vi "Derivative of intensity graph V1.2.vi"() -> ()   [LabVIEW 2016] (continued)
  in  "stop viewing ?":bool
  out "Y index 2":dbl=103.0
  in  "Pause viewing ?":bool
  in  "Decimate index":dbl=1.0
  in  "Name":T3={"X"="Vsd (V)", "Y"="VsgL (V)", "Z"="I (A)", "dZ/dX"="dI/dV (S)"}
  in  "Enum":T4(ring)=enum."dz/dx vs x"
  out "Derivative of Data":dbl[][](graph)
  out "Column number":i32=1229
  out "Row number":i32=321
  out "Ex":T5={"Offset"=-0.1923, "Multiplier"=0.0004} {"Offset" format="%#_6p"; "Multiplier" format="%#_6p"}
  in  "Ey":T5={"Offset"=-0.8, "Multiplier"=0.005}
  out "Data":dbl[][](graph)
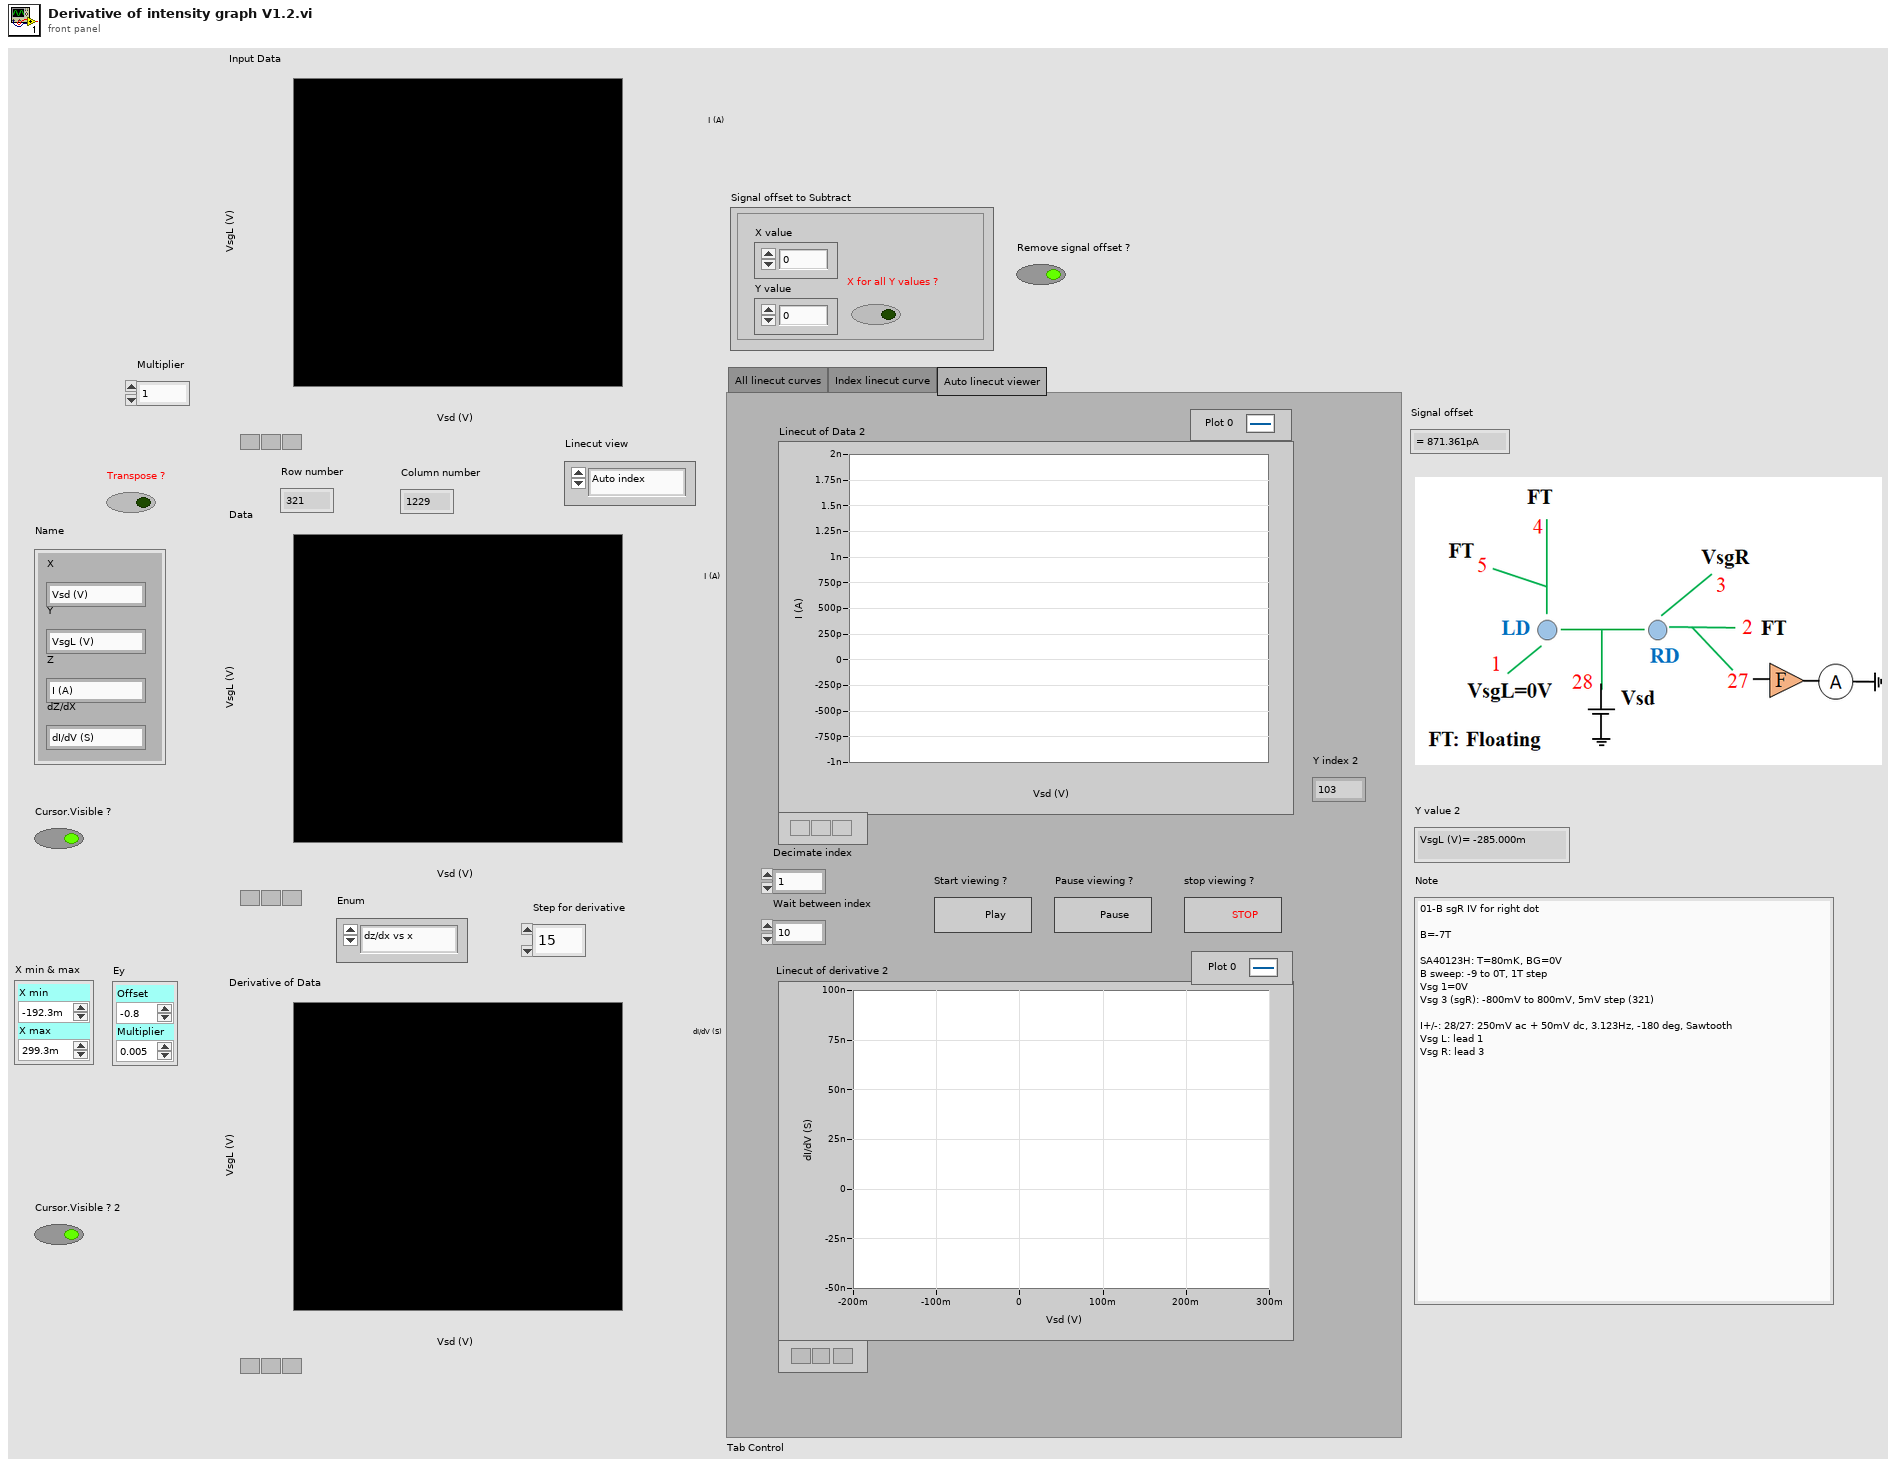
[diagram p1: front panel]
types:
  T1 = cluster{"X value":dbl, "Y value":dbl, "X for all Y values ?":bool}
  T2 = enum32{"All linecut curves", "Index linecut curve", "Auto linecut viewer"}
  T3 = cluster{"X":string, "Y":string, "Z":string, "dZ/dX":string}
  T4 = enum16{"dz/dx vs z", "dz/dx vs x", "dx/dz vs z", "dx/dz vs x"}
  T5 = typedef "LVOffsetAndMultiplierTypeDef.ctl" = cluster{"Offset":dbl, "Multiplier":dbl}
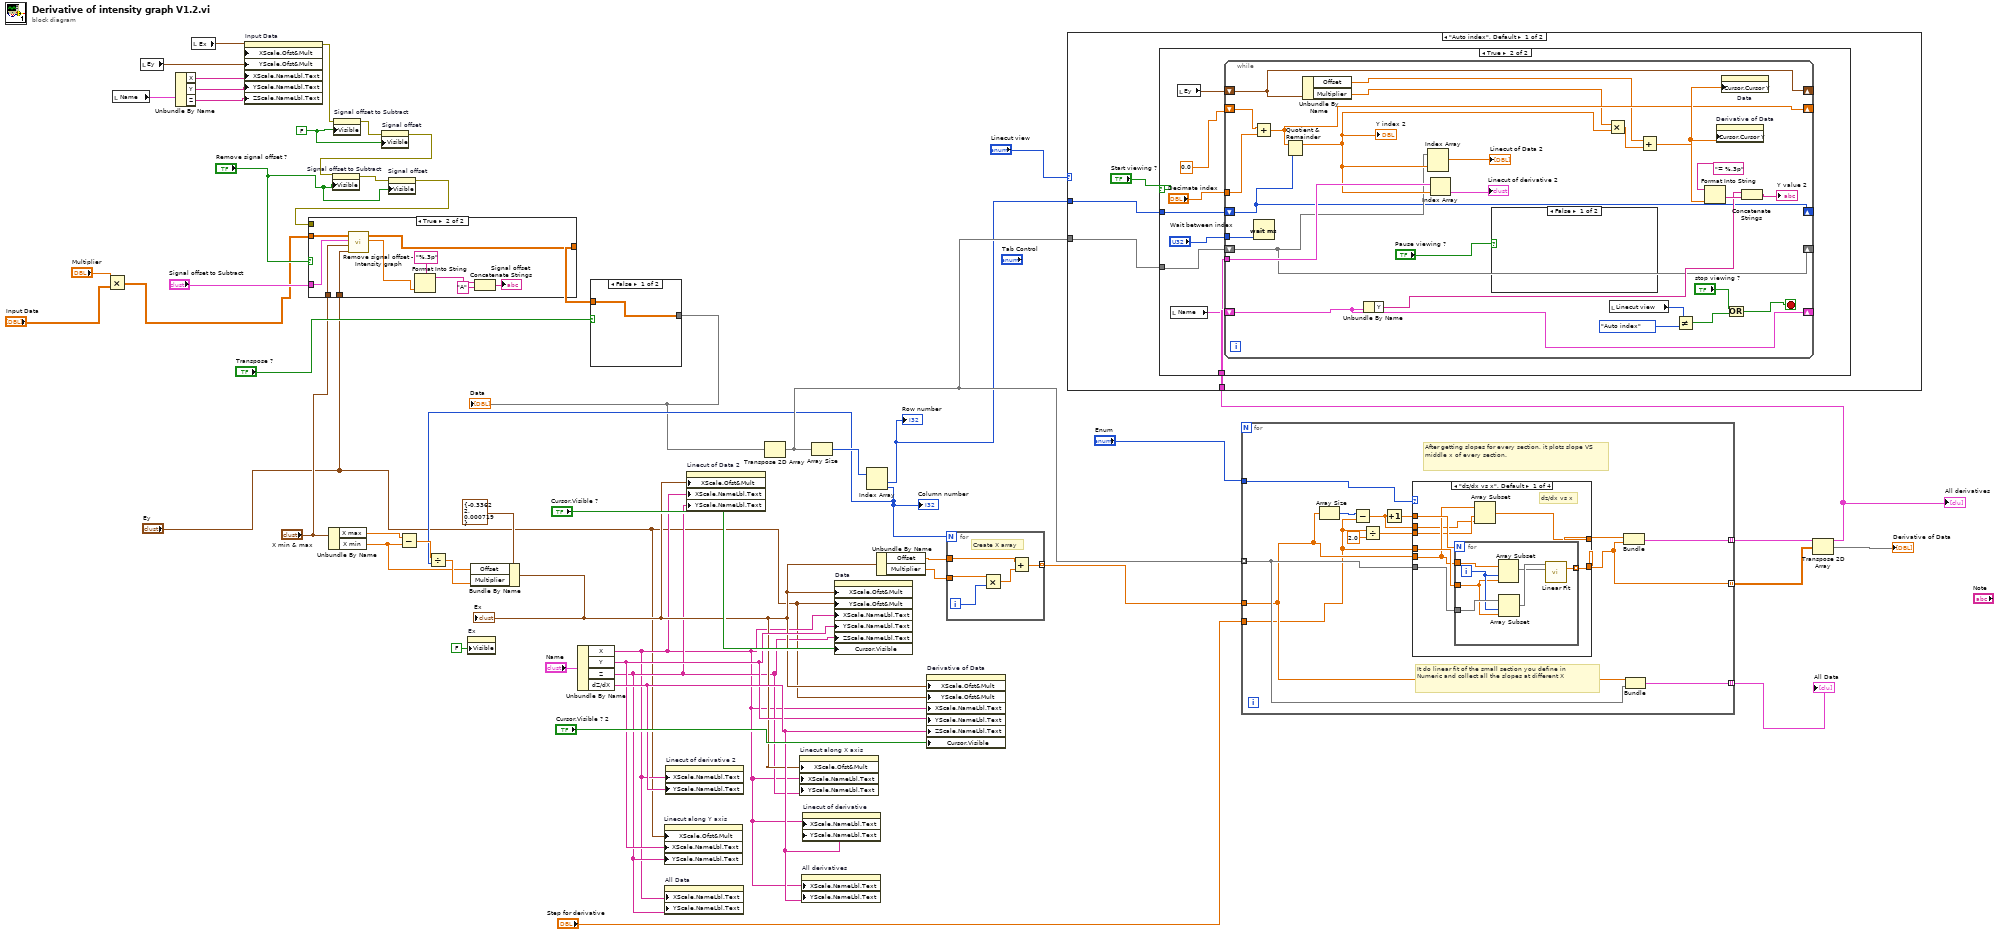
[diagram p0: block diagram]
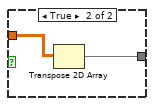
[diagram p3: hidden frame]
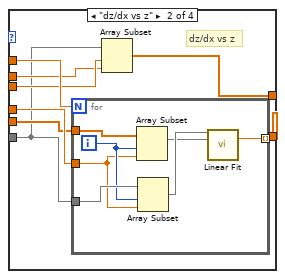
[diagram p4: hidden frame]
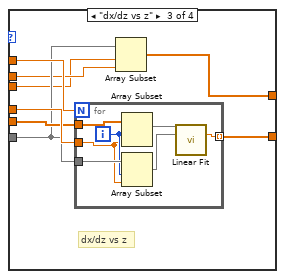
[diagram p5: hidden frame]
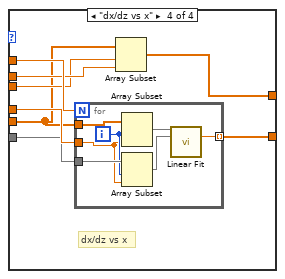
[diagram p6: hidden frame]
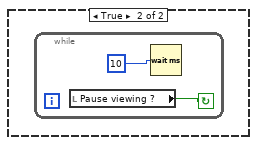
[diagram p8: hidden frame]
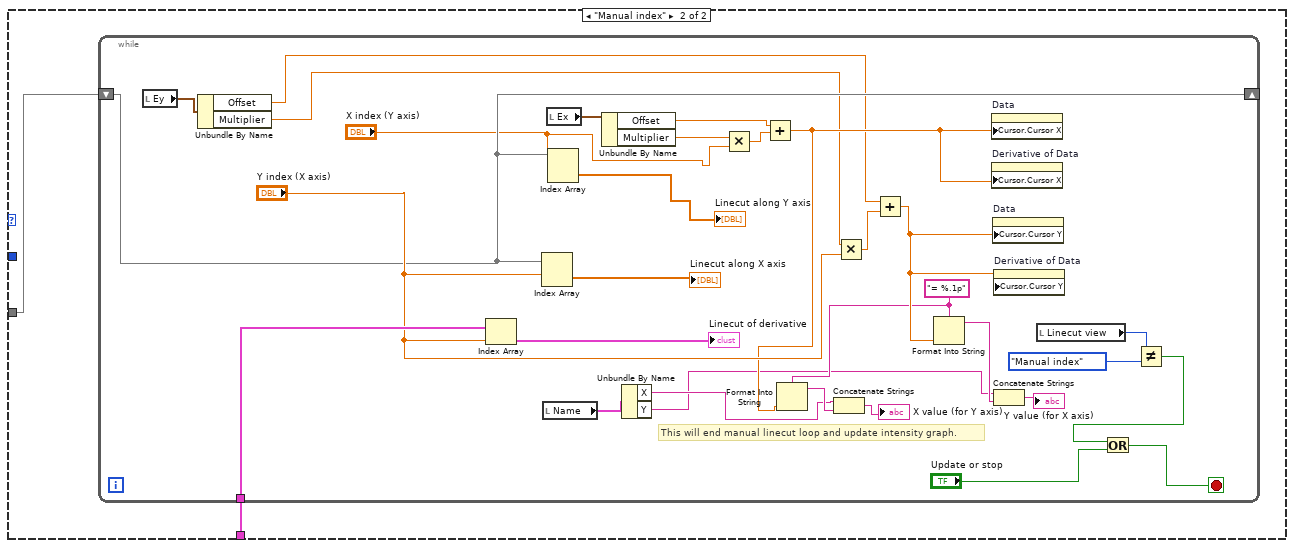
[diagram p9: hidden frame]
diagram:
  w14 = FALSE ("Visible")
  n1 = Multiply(x="Multiplier", y="Input Data") -> (x*y=w3:dbl[][])
  n2 = local read "Name"() -> (w19:T3)
  n3 = local read "Ey"() -> (w8:T5)
  n4 = Unbundle By Name(w19) -> ("X"=w18:string, "Y"=w17:string, "Z"=w16:string)
  n5 = local read "Ex"() -> (w7:T5)
  n6 = property on="Input Data" class="IntGraph (strict)"("XScale.Ofst&Mult"=w7, "YScale.Ofst&Mult"=w8, "XScale.NameLbl.Text"=w18, "YScale.NameLbl.Text"=w17, "ZScale.NameLbl.Text"=w16) -> (error out=w15:errorcluster)  [unwired: 2 in, 1 out]
  n7 = Unbundle By Name("X min & max") -> ("X max"=w32:dbl, "X min"=w27:dbl)
  n8 = property on="Signal offset to Subtract" class="Clust (strict)"(error in=w15, "Visible"=w14) -> (error out=w13:errorcluster)  [unwired: 1 in, 1 out]
  n9 = property on="Signal offset" class="Str"(error in=w13, "Visible"=w14) -> (error out=w12:errorcluster)  [unwired: 1 in, 1 out]
  n10 = property on="Signal offset to Subtract" class="Clust (strict)"(error in=w12, "Visible"="Remove signal offset ?") -> (error out=w10:errorcluster)  [unwired: 1 in, 1 out]
  n11 = property on="Signal offset" class="Str"(error in=w10, "Visible"="Remove signal offset ?") -> (error out=w9:errorcluster)  [unwired: 1 in, 1 out]
  n12 = case shown="True" "Remove signal offset ?" {
    tunnel: w3 -> [w51 w61]
    tunnel: [w51 w60] -> w21
    tunnel: "X min & max" -> [_ w58]
    tunnel: w9 -> [_ _]
    tunnel: "Signal offset to Subtract" -> [_ w59]
    tunnel: "Ey" -> [_ w57]
    frame False {
    }
    frame True {
      n13 = call "Remove signal offset - Intensity graph.vi"("Y Scale.Offset and Multiplier"=w57, "X min & max"=w58, "Current offset to Subtract"=w59, "Data"=w61) -> ("element"=w56:dbl, "Data 2"=w60:dbl[][])  [unwired: 6 in]
      n14 = Format Into String(format string="%.3p", w56) -> (resulting string=w54:string)  [unwired: 2 in, 1 out]
      n15 = Concatenate Strings(w54, "A" ("string")) -> (→"Signal offset":string)
    }
  }
  n16 = Subtract(x=w32, y=w27) -> (x-y=w30:dbl)
  n17 = property on="Ex" class="Clust (strict)"("Visible"=FALSE) -> ()  [unwired: 2 in, 2 out]
  n18 = Unbundle By Name("Name") -> ("X"=w22:string, "Y"=w33:string, "Z"=w23:string, "dZ/dX"=w34:string)
  n19 = case shown="False" "Transpose ?" {
    tunnel: w21 -> [w62 w64]
    tunnel: [w62 w63] -> w1
    frame False {
    }
    frame True {
      n20 = Transpose 2D Array(2D array=w64) -> (transposed array=w63:dbl[][])
    }
  }
  "Data" <- w1
  n21 = property on="Linecut along Y axis" class="WFGraph (strict)"("XScale.Ofst&Mult"="Ey", "XScale.NameLbl.Text"=w33, "YScale.NameLbl.Text"=w23) -> ()  [unwired: 2 in, 2 out]
  n22 = property on="All Data" class="XYGraph (strict)"("XScale.NameLbl.Text"=w22, "YScale.NameLbl.Text"=w23) -> ()  [unwired: 2 in, 2 out]
  n23 = property on="Linecut of derivative 2" class="XYGraph (strict)"("XScale.NameLbl.Text"=w22, "YScale.NameLbl.Text"=w34) -> ()  [unwired: 2 in, 2 out]
  n24 = Transpose 2D Array(2D array=w1) -> (transposed array=w37:dbl[][])
  n25 = property on="All derivatives" class="XYGraph (strict)"("XScale.NameLbl.Text"=w22, "YScale.NameLbl.Text"=w34) -> ()  [unwired: 2 in, 2 out]
  n26 = property on="Linecut of derivative" class="XYGraph (strict)"("XScale.NameLbl.Text"=w22, "YScale.NameLbl.Text"=w34) -> ()  [unwired: 2 in, 2 out]
  n27 = Array Size(array=w37) -> (size(s)=w46:i32[])
  n28 = Index Array(array=w46) -> (element #1=w36:i32, element #2=w29:i32)  [unwired: 2 in]
  "Row number" <- w36
  "Column number" <- w29
  n29 = Divide(x=w30, y=w29) -> (x/y=w28:dbl)
  n30 = Bundle By Name(cluster=T5 {"Offset"=-0.33622, "Multiplier"=0.000719} ("Ex"), "Offset"=w27, "Multiplier"=w28) -> (w26:T5)
  "Ex" <- w26
  n31 = property on="Linecut of Data 2" class="WFGraph (strict)"("XScale.Ofst&Mult"=w26, "XScale.NameLbl.Text"=w22, "YScale.NameLbl.Text"=w23) -> ()  [unwired: 2 in, 2 out]
  n32 = property on="Linecut along X axis" class="WFGraph (strict)"("XScale.Ofst&Mult"=w26, "XScale.NameLbl.Text"=w22, "YScale.NameLbl.Text"=w23) -> ()  [unwired: 2 in, 2 out]
  n33 = property on="Data" class="IntGraph (strict)"("XScale.Ofst&Mult"=w26, "YScale.Ofst&Mult"="Ey", "XScale.NameLbl.Text"=w22, "YScale.NameLbl.Text"=w33, "ZScale.NameLbl.Text"=w23, "Cursor.Visible"="Cursor.Visible ?") -> ()  [unwired: 2 in, 2 out]
  n34 = Unbundle By Name(w26) -> ("Offset"=w44:dbl, "Multiplier"=w45:dbl)
  n35 = property on="Derivative of Data" class="IntGraph (strict)"("XScale.Ofst&Mult"=w26, "YScale.Ofst&Mult"="Ey", "XScale.NameLbl.Text"=w22, "YScale.NameLbl.Text"=w33, "ZScale.NameLbl.Text"=w34, "Cursor.Visible"="Cursor.Visible ? 2") -> ()  [unwired: 2 in, 2 out]
  n36 = for {
    N: w29 -> [_]
    tunnel: w45 -> [w69]
    tunnel: w44 -> [w67]
    tunnel: [w65] -> w43 mode=indexing
    i -> [w68]
    # "Create X array"
    n37 = Multiply(x=w69, y=w68) -> (x*y=w66:dbl)
    n38 = Add(x=w67, y=w66) -> (x+y=w65:dbl)
  }
  n39 = for {
    tunnel: [w77] -> w38 mode=indexing
    tunnel: "Enum" -> [w76]
    tunnel: w43 -> [w72]
    tunnel: w37 -> [w73] mode=indexing
    tunnel: [w74] -> w40 mode=indexing
    tunnel: [w71] -> w39 mode=indexing
    tunnel: "Step for derivative" -> [w70]
    # "After getting slopes for every section, it plots slope VS middle x of every section."
    # "It do linear fit of the small section you define in Numeric and collect all the slopes at different X"
    n40 = Array Size(array=w72) -> (size(s)=w75:i32)
    n41 = Subtract(x=w75, y=w70) -> (x-y=w79:dbl)
    n42 = Divide(x=w70, y=2.0) -> (x/y=w80:dbl)
    n43 = Increment(x=w79) -> (x+1=w82:dbl)
    n44 = case shown="\"dz/dx vs x\", Default" w76 {
      tunnel: w82 -> [w90 w105 w120 w135]
      tunnel: w70 -> [w89 w104 w119 w134]
      tunnel: [w83 w99 w113 w129] -> w74
      tunnel: w72 -> [w87 w103 w118 w128]
      tunnel: w73 -> [w88 w98 w117 w133]
      tunnel: w80 -> [w86 w102 w115 w131]
      tunnel: w79 -> [w85 w101 w116 w132]
      tunnel: [w84 w100 w114 w130] -> w78
      frame "dz/dx vs x", Default {
        # "dz/dx vs x"
        n45 = for {
          N: w90 -> [_]
          tunnel: w87 -> [w97]
          tunnel: w88 -> [w96]
          tunnel: w89 -> [w94]
          tunnel: [w93] -> w83 mode=indexing
          i -> [w95]
          n46 = Array Subset(array=w97, index=w95, length=w94) -> (w91:dbl[])
          n47 = Array Subset(array=w96, index=w95, length=w94) -> (w92:dbl[])
          n48 = call <vilib>:"Linear Fit.vi"("Y"=w92, "X"=w91) -> ("slope"=w93:dbl)  [unwired: 9 in, 4 out]
        }
        n49 = Array Subset(array=w87, index=w86, length=w85) -> (w84:dbl[])
      }
      frame "dz/dx vs z" {
        # "dz/dx vs z"
        n50 = for {
          N: w105 -> [_]
          tunnel: w103 -> [w112]
          tunnel: w98 -> [w111]
          tunnel: w104 -> [w109]
          tunnel: [w108] -> w99 mode=indexing
          i -> [w110]
          n51 = Array Subset(array=w112, index=w110, length=w109) -> (w106:dbl[])
          n52 = Array Subset(array=w111, index=w110, length=w109) -> (w107:dbl[])
          n53 = call <vilib>:"Linear Fit.vi"("Y"=w107, "X"=w106) -> ("slope"=w108:dbl)  [unwired: 9 in, 4 out]
        }
        n54 = Array Subset(array=w98, index=w102, length=w101) -> (w100:dbl[])
      }
      frame "dx/dz vs z" {
        # "dx/dz vs z"
        n55 = for {
          N: w120 -> [_]
          tunnel: w118 -> [w127]
          tunnel: w117 -> [w126]
          tunnel: w119 -> [w124]
          tunnel: [w123] -> w113 mode=indexing
          i -> [w125]
          n56 = Array Subset(array=w127, index=w125, length=w124) -> (w122:dbl[])
          n57 = Array Subset(array=w126, index=w125, length=w124) -> (w121:dbl[])
          n58 = call <vilib>:"Linear Fit.vi"("Y"=w122, "X"=w121) -> ("slope"=w123:dbl)  [unwired: 9 in, 4 out]
        }
        n59 = Array Subset(array=w117, index=w115, length=w116) -> (w114:dbl[])
      }
      frame "dx/dz vs x" {
        # "dx/dz vs x"
        n60 = for {
          N: w135 -> [_]
          tunnel: w128 -> [w142]
          tunnel: w133 -> [w141]
          tunnel: w134 -> [w139]
          tunnel: [w138] -> w129 mode=indexing
          i -> [w140]
          n61 = Array Subset(array=w142, index=w140, length=w139) -> (w137:dbl[])
          n62 = Array Subset(array=w141, index=w140, length=w139) -> (w136:dbl[])
          n63 = call <vilib>:"Linear Fit.vi"("Y"=w137, "X"=w136) -> ("slope"=w138:dbl)  [unwired: 9 in, 4 out]
        }
        n64 = Array Subset(array=w128, index=w131, length=w132) -> (w130:dbl[])
      }
    }
    n65 = Bundle(w78, w74) -> (w77:cluster{dbl[], dbl[]})  [unwired: 1 in]
    n66 = Bundle(w72, w73) -> (w71:cluster{dbl[], dbl[]})  [unwired: 1 in]
  }
  "All derivatives" <- w38
  "All Data" <- w39
  n67 = case shown="\"Auto index\", Default" "Linecut view" {
    tunnel: w38 -> [w146 w184]
    tunnel: w37 -> [w145 w183]
    tunnel: w36 -> [w144 _]
    frame "Auto index", Default {
      n68 = case shown="True" "Start viewing ?" {
        tunnel: w146 -> [_ w154]
        tunnel: w145 -> [_ w150]
        tunnel: w144 -> [_ w152]
        frame False {
        }
        frame True {
          n69 = local read "Name"() -> (w147:T3)
          n70 = local read "Ey"() -> (w148:T5)
          n71 = while {
            tunnel: w154 -> [w173]
            shift-right: [w168] -> _
            shift-left: 0.0 ("Multiplier") -> [w169]
            tunnel: "Wait between index" -> [w171]
            tunnel: "Decimate index" -> [w167]
            shift-right: [w158] -> _
            shift-left: w148 -> [w158]
            shift-right: [w157] -> _
            shift-left: w147 -> [w157]
            shift-right: [w156] -> _
            shift-left: w150 -> [w156]
            shift-right: [w155] -> _
            shift-left: w152 -> [w155]
            stop <- w162 stop-if-true
            n72 = Add(x=w169, y=w167) -> (x+y=w168:dbl)
            n73 = Wait (ms)(milliseconds to wait=w171) -> ()  [unwired: 1 out]
            n74 = Quotient & Remainder(x=w168, y=w155) -> (x-y*floor(x/y)=w172:dbl)  [unwired: 1 out]
            "Y index 2" <- w172
            n75 = Unbundle By Name(w158) -> ("Offset"=w160:dbl, "Multiplier"=w159:dbl)
            n76 = Unbundle By Name(w157) -> ("Y"=w161:string)
            n77 = Index Array(array=w156, index (row)=w172) -> (element=→"Linecut of Data 2":dbl[])  [unwired: 1 in]
            n78 = Index Array(array=w173, index=w172) -> (element=→"Linecut of derivative 2":cluster{dbl[], dbl[]})
            n79 = case shown="False" "Pause viewing ?" {
              frame False {
              }
              frame True {
                n80 = while {
                  stop <- w181 continue-if-true
                  n81 = local read "Pause viewing ?"() -> (w181:bool)
                  n82 = Wait (ms)(milliseconds to wait=u32 10) -> ()  [unwired: 1 out]
                }
              }
            }
            n83 = Multiply(x=w159, y=w172) -> (x*y=w179:dbl)
            n84 = local read "Linecut view"() -> (w165:enum16{"Manual index", "Auto index"})
            n85 = Add(x=w160, y=w179) -> (x+y=w177:dbl)
            n86 = Not Equal?(x=w165, y=enum16{"Manual index", "Auto index"}."Auto index" ("Linecut view")) -> (x != y?=w164:bool)
            n87 = Format Into String(format string="= %.3p", w177) -> (resulting string=w175:string)  [unwired: 2 in, 1 out]
            n88 = property on="Derivative of Data" class="IntGraph (strict)"("Cursor.Cursor Y"=w177) -> ()  [unwired: 2 in, 2 out]
            n89 = property on="Data" class="IntGraph (strict)"("Cursor.Cursor Y"=w177) -> ()  [unwired: 2 in, 2 out]
            n90 = Or(x="stop viewing ?", y=w164) -> (x .or. y?=w162:bool)
            n91 = Concatenate Strings(w161, w175) -> (→"Y value 2":string)
          }
        }
      }
    }
    frame "Manual index" {
      n92 = while {
        tunnel: w184 -> [w208]
        shift-right: [w201] -> _
        shift-left: w183 -> [w201]
        stop <- w202 stop-if-true
        w193 = "= %.1p" ("format string")
        # "This will end manual linecut loop and update intensity graph."
        n93 = local read "Ey"() -> (w188:T5)
        n94 = Unbundle By Name(w188) -> ("Offset"=w186:dbl, "Multiplier"=w185:dbl)
        n95 = Index Array(array=w208, index="Y index (X axis)") -> (element=→"Linecut of derivative":cluster{dbl[], dbl[]})
        n96 = Index Array(array=w201, index (row)="Y index (X axis)") -> (element=→"Linecut along X axis":dbl[])  [unwired: 1 in]
        n97 = local read "Name"() -> (w190:T3)
        n98 = local read "Ex"() -> (w199:T5)
        n99 = Index Array(array=w201, index (col)="X index (Y axis)") -> (element=→"Linecut along Y axis":dbl[])  [unwired: 1 in]
        n100 = Unbundle By Name(w199) -> ("Offset"=w196:dbl, "Multiplier"=w197:dbl)
        n101 = Unbundle By Name(w190) -> ("X"=w189:string, "Y"=w187:string)
        n102 = Multiply(x=w197, y="X index (Y axis)") -> (x*y=w195:dbl)
        n103 = Add(x=w196, y=w195) -> (x+y=w194:dbl)
        n104 = Format Into String(format string=w193, w194) -> (resulting string=w192:string)  [unwired: 2 in, 1 out]
        n105 = Concatenate Strings(w189, w192) -> (→"X value (for Y axis)":string)
        n106 = Multiply(x=w185, y="Y index (X axis)") -> (x*y=w213:dbl)
        n107 = Add(x=w186, y=w213) -> (x+y=w211:dbl)
        n108 = Format Into String(format string=w193, w211) -> (resulting string=w210:string)  [unwired: 2 in, 1 out]
        n109 = property on="Data" class="IntGraph (strict)"("Cursor.Cursor X"=w194) -> ()  [unwired: 2 in, 2 out]
        n110 = property on="Derivative of Data" class="IntGraph (strict)"("Cursor.Cursor X"=w194) -> ()  [unwired: 2 in, 2 out]
        n111 = property on="Data" class="IntGraph (strict)"("Cursor.Cursor Y"=w211) -> ()  [unwired: 2 in, 2 out]
        n112 = property on="Derivative of Data" class="IntGraph (strict)"("Cursor.Cursor Y"=w211) -> ()  [unwired: 2 in, 2 out]
        n113 = Concatenate Strings(w187, w210) -> (→"Y value (for X axis)":string)
        n114 = local read "Linecut view"() -> (w206:enum16{"Manual index", "Auto index"})
        n115 = Not Equal?(x=w206, y=enum16{"Manual index", "Auto index"}."Manual index" ("Linecut view")) -> (x != y?=w204:bool)
        n116 = Or(x=w204, y="Update or stop") -> (x .or. y?=w202:bool)
      }
    }
  }
  n117 = Transpose 2D Array(2D array=w40) -> (transposed array=→"Derivative of Data":dbl[][])
